vi "Generate B-Vg scales.vi"() -> ()   [LabVIEW 2016]
panel:
  out "X":dbl[][](graph)
  out "Y":dbl[][](array[numeric])
  out "X":dbl[][](array[numeric])
  in  "Data":dbl[][](graph)=array180x1000[180000 elements]
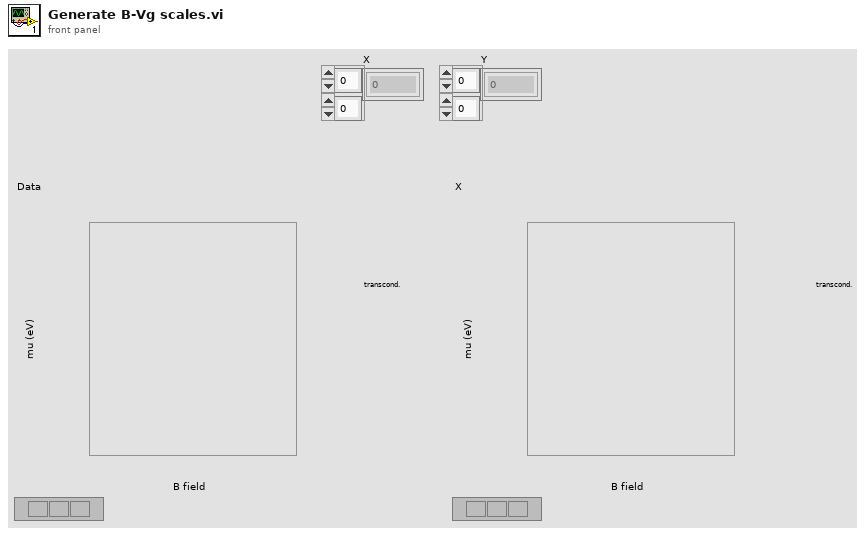
[diagram p1: front panel]
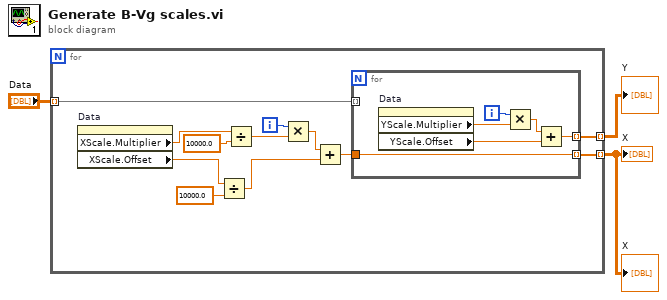
[diagram p0: block diagram]
diagram:
  n1 = for {
    tunnel: "Data" -> [w10] mode=indexing
    tunnel: [w12] -> w1 mode=indexing
    tunnel: [w11] -> w2 mode=indexing
    i -> [w15]
    n2 = property on="Data" class="IntGraph (strict)"() -> ("XScale.Multiplier"=w8:dbl, "XScale.Offset"=w5:dbl)  [unwired: 2 in, 2 out]
    n3 = Divide(x=w5, y=10000.0) -> (x/y=w4:dbl)
    n4 = Divide(x=w8, y=10000.0) -> (x/y=w7:dbl)
    n5 = Multiply(x=w15, y=w7) -> (x*y=w14:dbl)
    n6 = Add(x=w14, y=w4) -> (x+y=w13:dbl)
    n7 = for {
      tunnel: w13 -> [w17]
      tunnel: [w17] -> w12 mode=indexing
      tunnel: [w16] -> w11 mode=indexing
      tunnel: w10 -> [_] mode=indexing
      i -> [w20]
      n8 = property on="Data" class="IntGraph (strict)"() -> ("YScale.Multiplier"=w19:dbl, "YScale.Offset"=w18:dbl)  [unwired: 2 in, 2 out]
      n9 = Multiply(x=w20, y=w19) -> (x*y=w21:dbl)
      n10 = Add(x=w21, y=w18) -> (x+y=w16:dbl)
    }
  }
  "X" <- w1
  "Y" <- w2
  "X" <- w1
